vi "UHR-Fleezers Control (host) - 10.8MV_trial1.vi"() -> ()   [LabVIEW 2010] (continued)
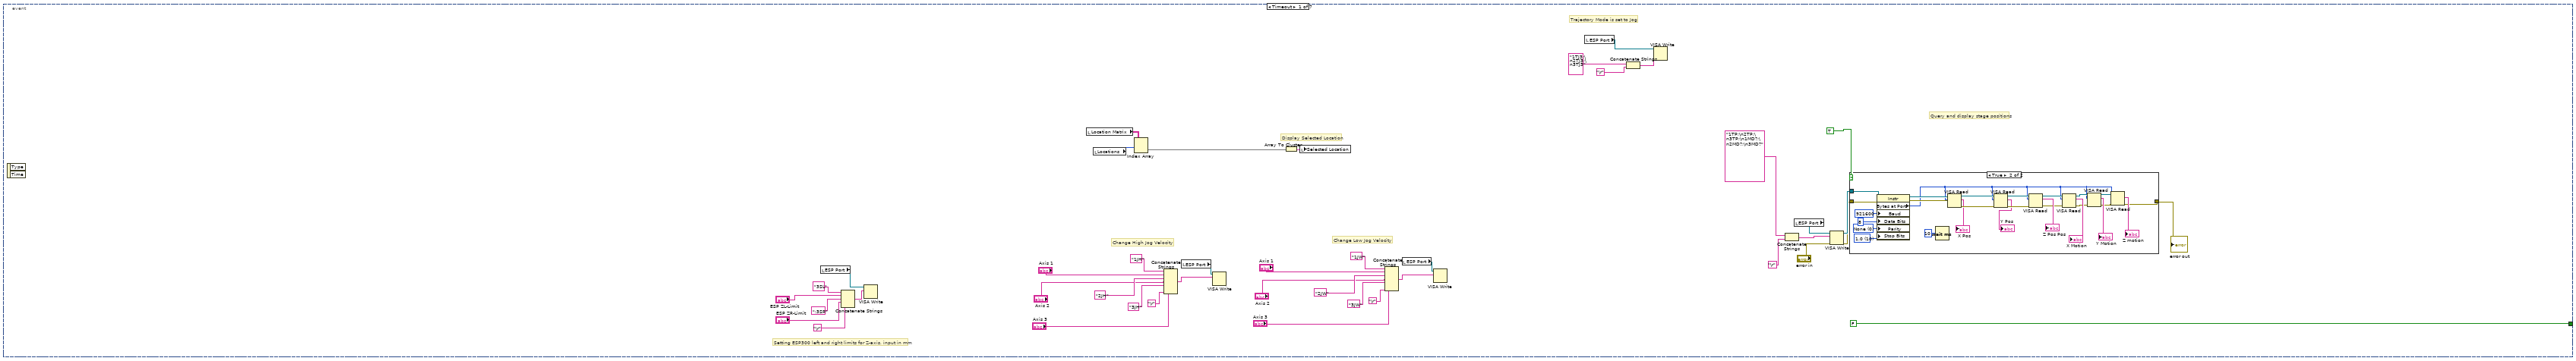
[diagram p2: hidden frame]
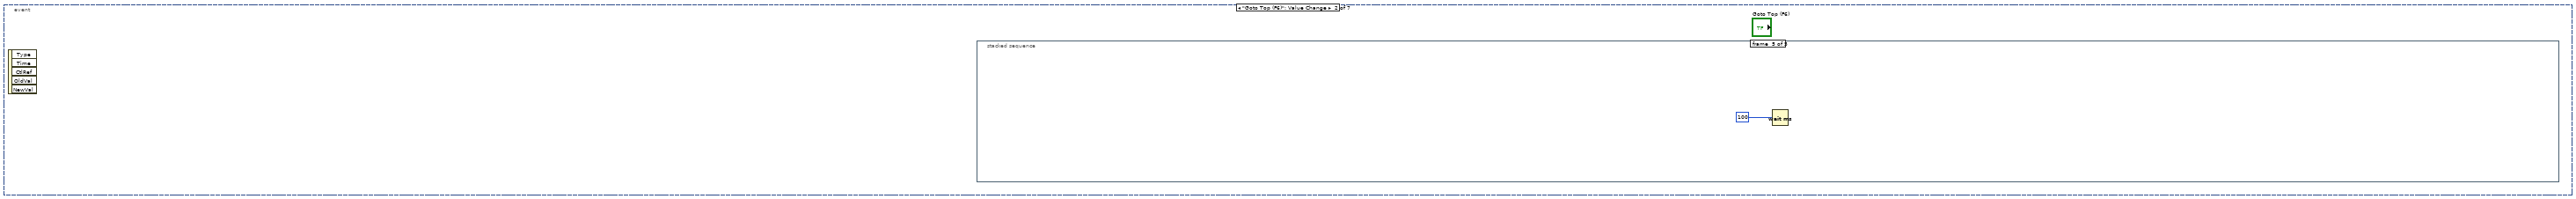
[diagram p4: hidden frame]
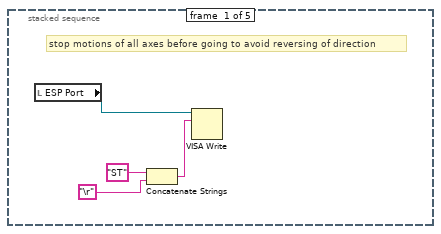
[diagram p5: hidden frame]
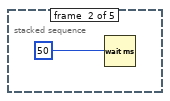
[diagram p6: hidden frame]
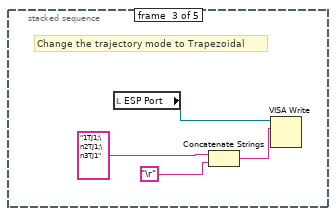
[diagram p7: hidden frame]
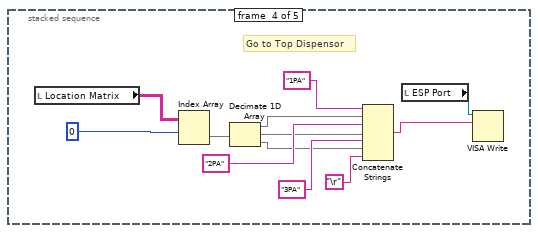
[diagram p8: hidden frame]
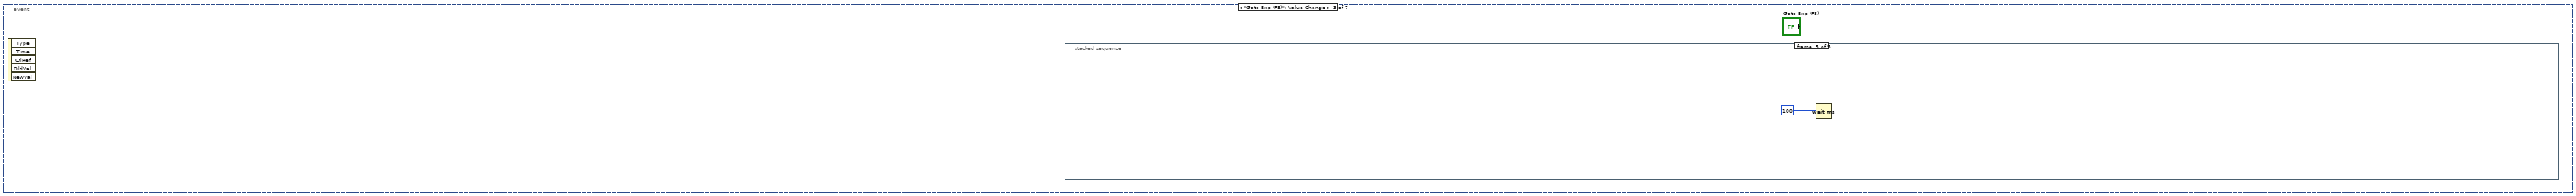
[diagram p9: hidden frame]
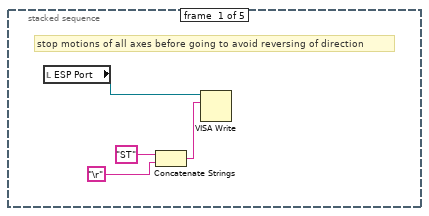
[diagram p10: hidden frame]
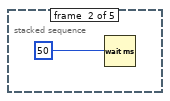
[diagram p11: hidden frame]
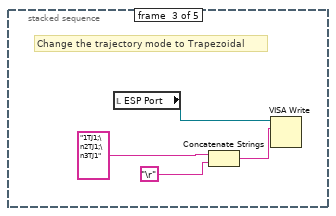
[diagram p12: hidden frame]
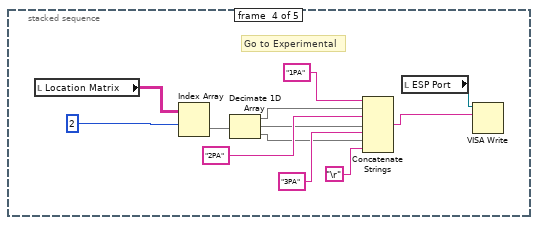
[diagram p13: hidden frame]
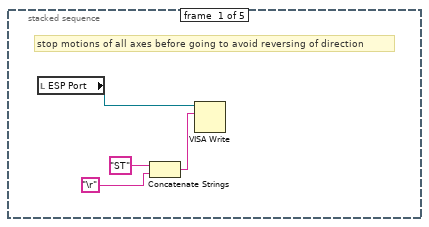
[diagram p14: hidden frame]
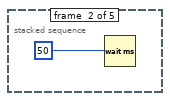
[diagram p15: hidden frame]
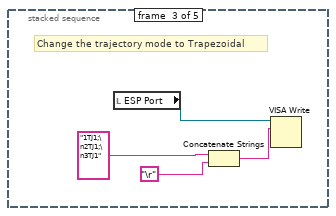
[diagram p16: hidden frame]
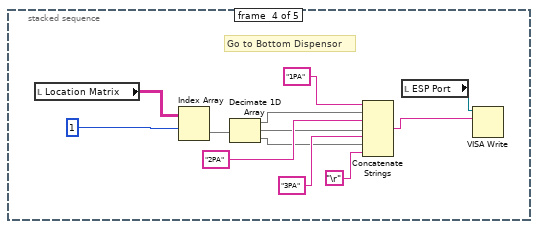
[diagram p17: hidden frame]
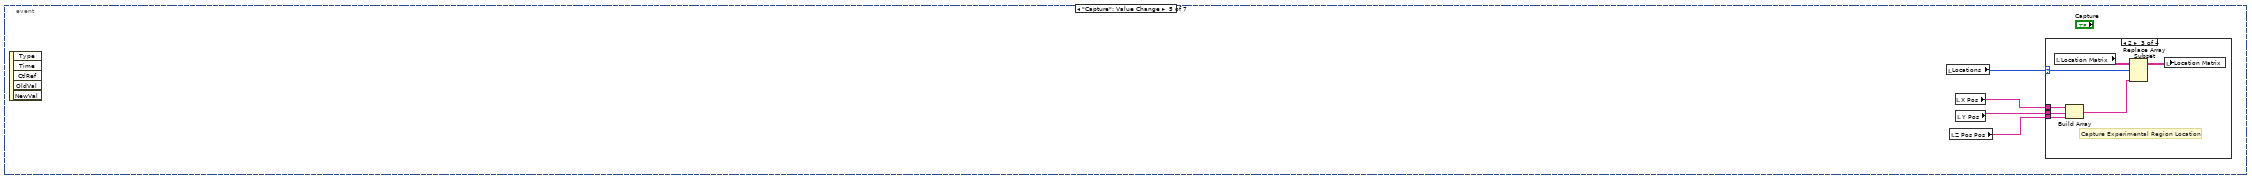
[diagram p18: hidden frame]
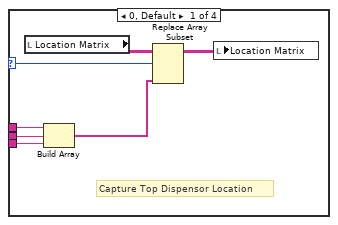
[diagram p19: hidden frame]
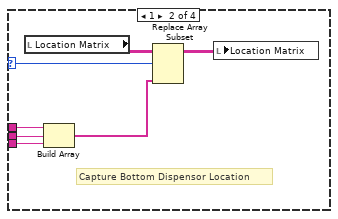
[diagram p20: hidden frame]
                n1978 = case shown="True" w8552 {
                  tunnel: w8553 -> [_ w8557]
                  frame False {
                  }
                  frame True {
                    n1979 = Close File(refnum=w8557) -> ()  [unwired: 1 in, 2 out]
                  }
                }
                n1980 = case shown="True" w8550 {
                  tunnel: w8551 -> [_ w8556]
                  frame False {
                  }
                  frame True {
                    n1981 = Close File(refnum=w8556) -> ()  [unwired: 1 in, 2 out]
                  }
                }
                n1982 = local write "Calibrating Trap..."(w8549) -> ()
                n1983 = call <vilib>:"Beep.vi"() -> ()  [unwired: 3 in, 9 out]
                n1984 = local write "Stop Saving"(w8549) -> ()
                n1985 = property on="Raster Scanning..." class="Bool (strict)"("Val(Sgnl)"=w8549) -> ()  [unwired: 2 in, 2 out]
                "Saving..." <- w8549
              }
              frame True {
                n1986 = local read "Calibrating Trap..."() -> (w8615:bool)
                n1987 = case "Write fl. data" shown="True" w8614 {
                  tunnel: w8613 -> [_ w8649]
                  tunnel: w8612 -> [_ w8648]
                  frame False {
                  }
                  frame True {
                    n1988 = Write to Binary File(file (use dialog)=w8649, data=w8648, 5:FALSE ("prepend array or string size? (T)"), 9:T31."big-endian, network order" ("byte order (0:big-endian, network order)")) -> ()  [unwired: 1 in, 4 out]
                  }
                }
                n1989 = Greater?(x="Save ave N", y=1.0) -> (0:w8618:bool)
                n1990 = Not(x=w8615) -> (.not. x?=w8617:bool)
                n1991 = And(x=w8617, y=w8618) -> (x .and. y?=w8560:bool)
                n1992 = case shown="True" w8560 {
                  tunnel: w8559 -> [w8629 w8640]
                  tunnel: [w8629 w8632] -> w8558
                  tunnel: "Save ave N" -> [_ w8633]
                  frame False {
                  }
                  frame True {
                    w8630 = 2 ("dimension size")
                    n1993 = Array Size(array=w8640) -> (size(s)=w8634:i32)
                    n1994 = Divide(x=w8634, y=w8630) -> (x/y=w8638:dbl)
                    n1995 = Reshape Array(w8640, w8638, w8630) -> (w8639:u64[][])
                    n1996 = Transpose 2D Array(2D array=w8639) -> (transposed array=w8637:u64[][])
                    n1997 = for {
                      tunnel: w8637 -> [w8642] mode=indexing
                      tunnel: [w8641] -> w8631 mode=indexing
                      tunnel: w8633 -> [w8643]
                      workers-P: _ -> [_]
                      n1998 = call "downsample 1D array - U64.vi"("Ave N"=w8643, "Array In"=w8642) -> ("Array Out"=w8641:u64[])  [unwired: 1 in]
                    }
                    n1999 = Transpose 2D Array(2D array=w8631) -> (transposed array=w8636:u64[][])
                    n2000 = Divide(x=w8634, y=w8633) -> (x/y=w8635:dbl)
                    n2001 = Reshape Array(w8636, w8635) -> (w8632:u64[])
                  }
                }
                n2002 = case shown="True" w8560 {
                  tunnel: w8620 -> [w8652 w8664]
                  tunnel: [w8652 w8656] -> w8616
                  tunnel: "Save ave N" -> [_ w8657]
                  tunnel: w8611 -> [_ w8655]
                  frame False {
                    # "don't downsample data for trap calibration"
                  }
                  frame True {
                    n2003 = Array Size(array=w8664) -> (size(s)=w8658:i32)
                    n2004 = Array Size(array=w8655) -> (size(s)=w8654:i32)
                    n2005 = Divide(x=w8658, y=w8654) -> (x/y=w8662:dbl)
                    n2006 = Reshape Array(w8664, w8662, w8654) -> (w8663:i16[][])
                    n2007 = Transpose 2D Array(2D array=w8663) -> (transposed array=w8661:i16[][])
                    n2008 = for {
                      tunnel: w8661 -> [w8667] mode=indexing
                      tunnel: [w8666] -> w8653 mode=indexing
                      tunnel: w8657 -> [w8665]
                      workers-P: _ -> [_]
                      n2009 = call "downsample 1D array - I16.vi"("Ave N"=w8665, "Array In"=w8667) -> ("Array Out"=w8666:i16[])  [unwired: 1 out]
                    }
                    n2010 = Transpose 2D Array(2D array=w8653) -> (transposed array=w8660:i16[][])
                    n2011 = Divide(x=w8658, y=w8657) -> (x/y=w8659:dbl)
                    n2012 = Reshape Array(w8660, w8659) -> (w8656:i16[])
                  }
                }
                n2013 = Index Array(array=w8582, index=1) -> (element=w8585:waveform(dbl))
                n2014 = Index Array(array=w8582, index=0) -> (element=w8587:waveform(dbl))
                n2015 = Unbundle By Name(w8585) -> ("Y"=w8589:dbl[])
                n2016 = Unbundle By Name(w8587) -> ("Y"=w8597:dbl[])
                n2017 = case "Write trap pos. data" shown="True" w8563 {
                  tunnel: w8562 -> [_ w8645]
                  tunnel: w8558 -> [_ w8644]
                  frame False {
                  }
                  frame True {
                    n2018 = Write to Binary File(file (use dialog)=w8645, data=w8644, 5:FALSE ("prepend array or string size? (T)"), 9:T31."big-endian, network order" ("byte order (0:big-endian, network order)")) -> ()  [unwired: 1 in, 4 out]
                  }
                }
                n2019 = Write to Binary File(file (use dialog)=w8623, data=w8616, 5:FALSE ("prepend array or string size? (T)"), 9:T31."big-endian, network order" ("byte order (0:big-endian, network order)")) -> ()  [unwired: 1 in, 4 out]
                n2020 = feedback #26(w8589) -> (w8591:dbl[])
                n2021 = Build Array (concatenate)(w8591, w8589) -> (w8590:dbl[])
                n2022 = Select(t=w8589, s=w8565, f=w8590) -> (s? t:f=w8575:dbl[])
                n2023 = feedback-in #26(w8575) -> ()
                n2024 = feedback #27(w8597) -> (w8610:dbl[])
                n2025 = Build Array (concatenate)(w8610, w8597) -> (w8609:dbl[])
                n2026 = Select(t=w8597, s=w8565, f=w8609) -> (s? t:f=w8584:dbl[])
                n2027 = feedback-in #27(w8584) -> ()
                n2028 = Divide(x=w8624, y=w8625) -> (x/y=w8627:dbl)
                n2029 = Multiply(x=w8627, y=100.0) -> (x*y=w8626:dbl)
                n2030 = Build Array(w8584, w8575) -> (→"Saved APD":dbl[][])
                n2031 = Array Size(array=w8584) -> (size(s)=w8602:i32)
                n2032 = Unbundle By Name(w8604) -> ("Y"=w8608:dbl[])
                n2033 = Subtract(x=w8602, y="N pts to average") -> (x-y=w8578:i32)
                n2034 = Multiply(x="N pts to average", y=u16 2) -> (x*y=w8579:u16)
                n2035 = Subtract(x=w8602, y=w8579) -> (x-y=w8577:i32)
                n2036 = feedback #28(w8608) -> (w8607:dbl[])
                n2037 = Build Array (concatenate)(w8607, w8608) -> (w8606:dbl[])
                n2038 = Select(t=w8608, s=w8565, f=w8606) -> (s? t:f=w8605:dbl[])
                "Trap Delta Graph" <- w8605
                n2039 = feedback-in #28(w8605) -> ()
                n2040 = Array Subset(array=w8584, index=w8578, length="N pts to average") -> (w8601:dbl[])
                n2041 = Array Subset(array=w8584, index=w8577, length="N pts to average") -> (w8600:dbl[])
                n2042 = Array Subset(array=w8575, index=w8578, length="N pts to average") -> (w8581:dbl[])
                n2043 = Array Subset(array=w8575, index=w8577, length="N pts to average") -> (w8580:dbl[])
                n2044 = call <vilib>:"Mean.vi"("X"=w8601) -> ("mean"=w8599:dbl)  [unwired: 1 out]
                n2045 = call <vilib>:"Mean.vi"("X"=w8581) -> ("mean"=w8574:dbl)  [unwired: 1 out]
                n2046 = call <vilib>:"Mean.vi"("X"=w8600) -> ("mean"=w8598:dbl)  [unwired: 1 out]
                n2047 = call <vilib>:"Mean.vi"("X"=w8580) -> ("mean"=w8573:dbl)  [unwired: 1 out]
                n2048 = Subtract(x=w8574, y=w8573) -> (x-y=w8564:dbl)
                "Delta Fl. 2" <- w8564
                n2049 = Subtract(x=w8599, y=w8598) -> (x-y=w8596:dbl)
                "Delta Fl. 1" <- w8596
                n2050 = Initialize Array(w8596, 1 ("dimension size")) -> (w8593:dbl[])
                n2051 = Initialize Array(w8564, 1 ("dimension size")) -> (w8570:dbl[])
                n2052 = feedback #29(w8593) -> (w8594:dbl[])
                n2053 = Build Array (concatenate)(w8594, w8593) -> (w8592:dbl[])
                n2054 = feedback #30(w8570) -> (w8571:dbl[])
                n2055 = Build Array (concatenate)(w8571, w8570) -> (w8569:dbl[])
                n2056 = Select(t=w8593, s=w8565, f=w8592) -> (s? t:f=w8568:dbl[])
                n2057 = feedback-in #29(w8568) -> ()
                n2058 = Select(t=w8570, s=w8565, f=w8569) -> (s? t:f=w8567:dbl[])
                n2059 = feedback-in #30(w8567) -> ()
                n2060 = Build Array(w8568, w8567) -> (→"Save APD Deriv":dbl[][])
              }
            }
            "Progress" <- w8541
            "Progress 2" <- w8541
          }
        }
      }
    }
    n2061 = Bundle By Name(cluster=w5584, "Green FB Ch 0"=w5583, "Green FB Ch 1"=w5582) -> (w5562:T50)
    "Green FB Signals (V)" <- w5562
    n2062 = Unbundle By Name(w5562) -> ("Green FB Ch 2"=→"Green FB Plot":dbl)
    n2063 = local read "wait to reset values"() -> (w5654:bool)
    n2064 = Not(x=w5651) -> (.not. x?=w5655:bool)
    n2065 = And(x=w5655, y=w5654) -> (x .and. y?=w5656:bool)
    n2066 = case "Part of MCL raster scanning: returns to initial positions after scan done" shown="True" w5656 {
      tunnel: w5659 -> [w7258 w7265]
      tunnel: [w7258 w7264] -> w5658
      tunnel: w5653 -> [w7257 w7263]
      tunnel: [w7257 w7262] -> w5652
      frame False {
      }
      frame True {
        w7273 = 10.0 ("y")
        w7272 = 32767.0 ("y")
        # "to return scan values\nafter a synchronous \nAOM scan"
        n2067 = local read "AO2"() -> (w7266:dbl)
        n2068 = local read "AO1"() -> (w7267:dbl)
        n2069 = local write "wait to reset values"(FALSE ("wait to reset values")) -> ()
        n2070 = Multiply(x=w7267, y=w7272) -> (x*y=w7269:dbl)
        n2071 = Multiply(x=w7266, y=w7272) -> (x*y=w7271:dbl)
        n2072 = Divide(x=w7269, y=w7273) -> (x/y=w7268:dbl)
        n2073 = Divide(x=w7271, y=w7273) -> (x/y=w7270:dbl)
        n2074 = To Word Integer(number=w7268) -> (16bit integer=w7274:i16)
        n2075 = To Word Integer(number=w7270) -> (16bit integer=w7275:i16)
        n2076 = local read "Total Counts (ticks)"() -> (w7259:u32)
        n2077 = xnode "Read/Write Control"("FPGA VI Reference In"=w7265, "error in"=w7263, "AO1"=w7274, "AO2"=w7275, "MCL count"=w7259) -> ("FPGA VI Reference Out"=w7264:T19, "error out"=w7262:errorcluster)
        n2078 = local read "Scan Range (V)\n(of steps)"() -> (w7260:dbl)
        n2079 = property on="Scan Range (V)\n(of steps)" class="DigNum (strict)"("Val(Sgnl)"=w7260) -> ()  [unwired: 2 in, 2 out]
      }
    }
    n2080 = node-c288() -> ()  [unwired: 2 out]
  }
  n2081 = node-c288(3 ("Processor")) -> (w74:T26)  [unwired: 3 out]
  n2082 = timed-loop "Oscillate AOD (debugging)" {
    tunnel: w24 -> [w8669]
    tunnel: [w8668] -> w36
    timing: w74 -> [_]
    timing-out: [_] -> w73
    stop <- w8668 stop-if-true
    n2083 = node-c288() -> ()  [unwired: 2 out]
    n2084 = event shown="[0] \"Oscillate Set 2\", \"Fish for Tether\": Value Change" {
      selector: _ -> [_ _ _]
      dyn-events: _ -> [_ _ _]
      timeout: _ -> [_ _ _]
      tunnel: w8669 -> [w8676 _ _]
      tunnel: [FALSE ("Stop All") _ w8944] -> w8668
      event "Oscillate Set 2", "Fish for Tether": Value Change {
        n2085 = event-data() -> ()  [unwired: 6 out]
        n2086 = local read "Oscillate Set 2"() -> (w8675:bool)
        n2087 = Or(x=w8675, y="Fish for Tether") -> (x .or. y?=w8673:bool)
        n2088 = case shown="True" w8673 {
          tunnel: w8676 -> [_ w8679]
          tunnel: "Fish for Tether" -> [_ w8678]
          frame False {
          }
          frame True {
            n2089 = case shown="True" w8678 {
              frame False {
              }
              frame True {
                n2090 = local write "Scan axis 2"(TRUE) -> ()
                n2091 = local write "Tether"(FALSE ("Tether")) -> ()
              }
            }
            n2092 = node-c288("Period") -> (w8681:T26)  [unwired: 3 out]
            n2093 = timed-loop "Oscillate AOD" {
              timing: w8681 -> [_]
              timing-out: [_] -> w8680
              tunnel: w8679 -> [w8691]
              tunnel: w8678 -> [w8690]
              i -> [w8693]
              stop <- w8689 stop-if-true
              n2094 = node-c288() -> (w8692:i64)  [unwired: 1 out]
              n2095 = flat-sequence {
                tunnel: w8693 -> [w8719]
                tunnel: w8692 -> [w8718]
                tunnel: w8691 -> [w8702]
                tunnel: w8690 -> [w8704]
                tunnel: [w8704] -> w8688
                tunnel: [w8703] -> w8687
                tunnel: [w8701] -> w8686
                tunnel: [w8698] -> w8684
                tunnel: w8688 -> [w8755]
                tunnel: w8687 -> [w8753]
                tunnel: w8686 -> [w8752]
                tunnel: [w8751] -> w8685
                tunnel: w8684 -> [w8750]
                tunnel: [w8819] -> w8689
                tunnel: w8685 -> [w8817]
                frame #0 {
                  n2096 = Divide(x=w8718, y=i64 1000) -> (x/y=w8713:dbl)
                  n2097 = Multiply(x=w8713, y=w8719) -> (x*y=w8715:dbl)
                  n2098 = Multiply(x="Osc. freq. (Hz)", y=6.283185307179586) -> (x*y=w8716:dbl)
                  n2099 = Multiply(x=w8716, y=w8715) -> (x*y=w8700:dbl)
                  n2100 = local read "BD 1 Frequency 2 (MHz)"() -> (w8697:dbl)
                  n2101 = local read "BD 1 Frequency 1 (MHz)"() -> (w8694:dbl)
                  n2102 = case shown="True" w8704 {
                    tunnel: w8700 -> [w8725 w8732]
                    tunnel: w8697 -> [_ w8742]
                    tunnel: [w8722 w8726] -> w8705
                    tunnel: [FALSE w8735] -> w8701
                    tunnel: [0.0 w8728] -> w8698
                    tunnel: w8694 -> [_ w8727]
                    frame False {
                      n2103 = Sine(x=w8725) -> (sin(x)=w8723:dbl)
                      n2104 = Multiply(x=w8723, y="Osc. amp. (MHz)") -> (x*y=w8722:dbl)
                    }
                    frame True {
                      n2105 = Cosine(x=w8732) -> (cos(x)=w8745:dbl)
                      n2106 = Subtract(x=w8742, y=w8727) -> (x-y=w8741:dbl)
                      n2107 = Decrement(x=w8745) -> (x-1=w8744:dbl)
                      n2108 = Subtract(x=w8741, y="Closest Delta (MHz)") -> (x-y=w8738:dbl)
                      n2109 = Divide(x=w8744, y=2.0) -> (x/y=w8739:dbl)
                      n2110 = Multiply(x=w8739, y=w8738) -> (x*y=w8726:dbl)
                      n2111 = local read "Vec Mean of T1 T2"() -> (w8734:dbl[])
                      n2112 = Greater?(x=w8734, y="Stop F (pN)") -> (0:w8736:bool[])
                      n2113 = Or Array Elements(Boolean array=w8736) -> (logical OR=w8735:bool)
                      n2114 = Divide(x=w8732, y=6.283185307179586) -> (x/y=w8731:dbl)
                      n2115 = Round Toward +Infinity(x=w8731) -> (ceil(x): smallest int >= x=w8728:dbl)
                      "Attempts" <- w8728
                      n2116 = Greater?(x=w8728, y="Attempt Limit") -> (0:w8730:bool)
                      n2117 = case shown="True" w8730 {
                        frame False {
                        }
                        frame True {
                          n2118 = local write "Fish for Tether"(FALSE ("Fish for Tether")) -> ()
                          n2119 = call <vilib>:"Beep.vi"() -> ()  [unwired: 3 in, 9 out]
                          n2120 = local read "Messages"() -> (w8747:string)
                          n2121 = call "Update messages.vi"("Message to add"="Tether fishing timeout." ("Messages"), "Old message string"=w8747) -> ("New message string"=→"Messages":string)
                        }
                      }
                    }
                  }
                  n2122 = local read "Y RF Frequency Limits (MHz)"() -> (w8706:T16)
                  n2123 = local read "X RF Frequency Limits (MHz)"() -> (w8707:T16)
                  n2124 = local read "BD 1 Frequency 3 (MHz)"() -> (w8712:dbl)
                  n2125 = local read "BD 2 Frequency 2 (MHz)"() -> (w8696:dbl)
                  n2126 = Select(t=w8697, s="Scan axis 2", f=w8696) -> (s? t:f=w8708:dbl)
                  n2127 = Add(x=w8705, y=w8708) -> (x+y=w8703:dbl)
                  n2128 = Select(t=w8703, s="Scan axis 2", f=w8697) -> (s? t:f=w8695:dbl)
                  n2129 = Select(t=w8696, s="Scan axis 2", f=w8703) -> (s? t:f=w8710:dbl)
                  n2130 = local read "BD 2 Frequency 3 (MHz)"() -> (w8711:dbl)
                  n2131 = call "set RF board frequency - interlace.vi"("Board 2 Frequency Limits"=w8706, "Board 1 Frequency Limits"=w8707, "FPGA VI Reference In"=w8702, "Board 2 Frequency 3 (MHz)"=w8711, "Board 1 Frequency 3 (MHz)"=w8712, "Board 2 Frequency 2 (MHz)"=w8696, "Board 2 Frequency 1 (MHz)"=w8710, "Board 1 Frequency 2 (MHz)"=w8695, "Board 1 Frequency 1  (MHz)"=w8694) -> ()  [unwired: 1 in, 2 out]
                }
                frame #1 {
                  n2132 = And(x=w8755, y=w8752) -> (x .and. y?=w8754:bool)
                  n2133 = case "Only if were fishing and now formed tether" shown="True" w8754 {
                    tunnel: w8753 -> [w8757 w8769]
                    tunnel: [w8756 w8768] -> w8751
                    tunnel: w8750 -> [_ w8764]
                    frame False {
                      n2134 = local read "Fish for Tether"() -> (w8756:bool)
                      n2135 = case shown="True" w8756 {
                        tunnel: w8757 -> [_ _]
                        frame False {
                        }
                        frame True {
                        }
                      }
                    }
                    frame True {
                      w8768 = FALSE ("Fish for Tether")
                      n2136 = call <vilib>:"Beep.vi"() -> ()  [unwired: 3 in, 9 out]
                      n2137 = Number To Decimal String(number=w8764, width (-)=i16 1) -> (decimal integer string=w8762:string)
                      n2138 = case shown="\"2\", \"3\", \"4\", \"5\", \"6\"" "Then..." {
                        selector: "Then..." -> [_ w8772]
                        tunnel: w8769 -> [w8771 _]
                        frame "1", Default {
                          # "do nothing"
                          n2139 = property on="BD 1 Frequency 1 (MHz)" class="DigNum (strict)"("Val(Sgnl)"=w8771) -> ()  [unwired: 2 in, 2 out]
                        }
                        frame "2", "3", "4", "5", "6" {
                          n2140 = flat-sequence {
                            tunnel: w8772 -> [w8774]
                            frame #0 {
                              n2141 = property on="Trap Delta (MHz)" class="DigNum (strict)"("Val(Sgnl)"="Move to Delta 1 (MHz)") -> ()  [unwired: 2 in, 2 out]
                            }
                            frame #1 {
                              n2142 = case shown="\"5\", \"6\"" w8774 {
                                selector: w8774 -> [w8777 w8787 _]
                                frame "3", "4" {
                                n2143 = flat-sequence {
                                tunnel: w8777 -> [w8778]
                                tunnel: [w8778] -> w8775
                                tunnel: [w8780] -> w8776
                                tunnel: w8775 -> [w8780]
                                tunnel: w8776 -> [w8784]
                                frame #0 {
                                n2144 = property on="Green Laser ON/Interlacing" class="Bool (strict)"("Val(Sgnl)"=TRUE ("Value (Signaling)")) -> ()  [unwired: 2 in, 2 out]
                                }
                                frame #1 {
                                n2145 = Multiply(x="Wait Before Save (s)", y=u32 1000 ("x")) -> (x*y=w8782:u32)
                                n2146 = Wait (ms)(milliseconds to wait=w8782) -> ()  [unwired: 1 out]
                                }
                                frame #2 {
                                n2147 = property on="Start Saving" class="Bool (strict)"("Value"=TRUE ("Start Saving")) -> ()  [unwired: 2 in, 2 out]
                                n2148 = case shown="Default" w8784 {
                                frame Default {
                                }
                                frame "4" {
                                n2149 = property on="Fl. Triggered..." class="Bool (strict)"("Val(Sgnl)"=TRUE ("Value (Signaling)")) -> ()  [unwired: 2 in, 2 out]
                                }
                                }
                                }
                                }
                                }
                                frame "5", "6" {
                                n2150 = stacked-sequence {
                                tunnel: w8787 -> [_ _ _ _ _ _ _ _ w8804 _ _]
                                frame #0 {
                                n2151 = Replace Array Subset(array=u32[] [0] ("Index Values"), new element="Raster Set Upon Tether", index=0) -> (w8788:u32[])
                                n2152 = property on="Saved AOD Raster Scan Parameter Sets" class="Arr (strict)"("Index Values"=w8788) -> ()  [unwired: 2 in, 2 out]
                                }
                                frame #1 {
                                n2153 = Wait (ms)(milliseconds to wait=u32 500) -> ()  [unwired: 1 out]
                                }
                                frame #2 {
                                n2154 = property on="Load parameters" class="Bool (strict)"("Val(Sgnl)"=TRUE ("Value (Signaling)")) -> ()  [unwired: 2 in, 2 out]
                                }
                                frame #3 {
                                n2155 = Wait (ms)(milliseconds to wait=u32 500) -> ()  [unwired: 1 out]
                                }
                                frame #4 {
                                n2156 = property on="Trap Raster Scan" class="Bool (strict)"("Val(Sgnl)"=TRUE ("Value (Signaling)")) -> ()  [unwired: 2 in, 2 out]
                                }
                                frame #5 {
                                n2157 = Wait (ms)(milliseconds to wait=u32 2000) -> ()  [unwired: 1 out]
                                }
                                frame #6 {
                                n2158 = while {
                                stop <- w8799 stop-if-true
                                n2159 = local read "Raster Scanning..."() -> (w8798:bool)
                                n2160 = local read "Saving..."() -> (w8801:bool)
                                n2161 = Wait (ms)(milliseconds to wait=u32 100) -> ()  [unwired: 1 out]
                                n2162 = Not(x=w8801) -> (.not. x?=w8800:bool)
                                n2163 = Not(x=w8798) -> (.not. x?=w8797:bool)
                                n2164 = And(x=w8800, y=w8797) -> (x .and. y?=w8799:bool)
                                }
                                }
                                frame #7 {
                                n2165 = property on="Trap Delta (MHz)" class="DigNum (strict)"("Val(Sgnl)"="Move to Delta 2 (MHz)") -> ()  [unwired: 2 in, 2 out]
                                }
                                frame #8 {
                                n2166 = local read "Tether"() -> (w8805:bool)
                                n2167 = case shown="True" w8805 {
                                tunnel: w8804 -> [_ w8806]
                                frame False {
                                }
                                frame True {
                                n2168 = flat-sequence {
                                tunnel: w8806 -> [w8808]
                                frame #0 {
                                n2169 = Wait (ms)(milliseconds to wait=u32 500) -> ()  [unwired: 1 out]
                                }
                                frame #1 {
                                n2170 = case shown="\"6\"" w8808 {
                                frame Default {
                                }
                                frame "6" {
                                n2171 = property on="Green Laser ON/Interlacing" class="Bool (strict)"("Val(Sgnl)"=TRUE ("Green Laser ON/Interlacing")) -> ()  [unwired: 2 in, 2 out]
                                }
                                }
                                }
                                frame #2 {
                                n2172 = Wait (ms)(milliseconds to wait=u32 500) -> ()  [unwired: 1 out]
                                }
                                frame #3 {
                                n2173 = local write "Start Saving"("Save at end (5, 6)") -> ()
                                }
                                }
                                }
                                }
                                }
                                frame #9 {
                                n2174 = local read "Bead Sep. Int. Time (s)"() -> (w8814:dbl)
                                n2175 = Multiply(x=w8814, y=1000.0) -> (x*y=w8813:dbl)
                                n2176 = Wait (ms)(milliseconds to wait=w8813) -> ()  [unwired: 1 out]
                                }
                                frame #10 {
                                n2177 = property on="Rescale on Mean" class="Bool (strict)"("Val(Sgnl)"=TRUE ("Value (Signaling)")) -> ()  [unwired: 2 in, 2 out]
                                }
                                }
                                }
                                frame "2", Default {
                                }
                              }
                            }
                          }
                        }
                      }
                      n2178 = Concatenate Strings("Formed tether in ", w8762, " attempt(s)." ("string")) -> (w8759:string)
                      n2179 = local read "Messages"() -> (w8766:string)
                      n2180 = local write "Fish for Tether"(w8768) -> ()
                      n2181 = call "Update messages.vi"("Message to add"=w8759, "Old message string"=w8766) -> ("New message string"=w8765:string)
                      n2182 = local write "Messages"(w8765) -> ()
                      n2183 = Get Date/Time In Seconds() -> (seconds since 1Jan1904=→"Time tether formed":timestamp)
                      "Tether" <- "Tether Alarm?"
                    }
                  }
                }
                frame #2 {
                  n2184 = local read "Oscillate Set 2"() -> (w8818:bool)
                  n2185 = local read "Stop All"() -> (w8820:bool)
                  n2186 = Not Or(1:w8817, 2:w8818) -> (0:w8816:bool)
                  n2187 = Compound Arithmetic op=OR(w8820, w8816) -> (w8819:bool)
                }
              }
              n2188 = node-c288() -> ()  [unwired: 2 out]
            }
            n2189 = node-c288(w8680) -> ()  [unwired: 1 out]
          }
        }
      }
      event "Fl. Triggered...": Value Change {
        n2190 = event-data() -> ()  [unwired: 7 out]
        n2191 = case shown="True" "Fl. Triggered..." {
          frame False {
          }
          frame True {
            n2192 = node-c288() -> (w8832:T26)  [unwired: 4 out]
            n2193 = timed-loop {
              timing: w8832 -> [_]
              timing-out: [_] -> w8831
              tunnel: "Action" -> [w8836]
              shift-right: [w8833] -> _
              shift-left: u8 255 -> [w8835]
              stop <- w8837 stop-if-true
              n2194 = node-c288() -> ()  [unwired: 2 out]
              n2195 = flat-sequence {
                tunnel: w8836 -> [w8849]
                tunnel: w8835 -> [w8846]
                tunnel: [w8845] -> w8834
                tunnel: [w8935] -> w8837
                tunnel: w8834 -> [w8934]
                tunnel: [w8934] -> w8833
                frame #0 {
                  n2196 = local read "Delta Fl. 2"() -> (w8840:dbl)
                  n2197 = local read "Delta Fl. 1"() -> (w8841:dbl)
                  n2198 = Select(t=w8841, s="APD to Watch", f=w8840) -> (s? t:f=w8839:dbl)
                  n2199 = Multiply(x="Fl. Delta Thresh. (kHz)", y=1000.0) -> (x*y=w8848:dbl)
                  n2200 = Greater?(x=w8839, y=w8848) -> (0:w8843:bool)
                  n2201 = Or(x="Force Yank", y=w8843) -> (x .or. y?=w8844:bool)
                  n2202 = case shown="True" w8844 {
                    tunnel: w8849 -> [_ w8859]
                    tunnel: w8846 -> [w8851 w8855]
                    tunnel: [w8851 w8852] -> w8845
                    frame False {
                    }
                    frame True {
                      n2203 = flat-sequence {
                        tunnel: w8856 -> [w8865]
                        tunnel: [w8865] -> w8860
                        tunnel: w8859 -> [w8864]
                        tunnel: [w8864] -> w8858
                        tunnel: [w8863] -> w8857
                        tunnel: w8855 -> [w8862]
                        tunnel: [w8861] -> w8854
                        tunnel: w8860 -> [w8890]
                        tunnel: w8858 -> [w8889]
                        tunnel: w8857 -> [w8888]
                        tunnel: w8854 -> [w8887]
                        tunnel: [w8887] -> w8853
                        tunnel: w8853 -> [w8932]
                        tunnel: [w8932] -> w8852
                        frame #0 {
                          n2204 = call <vilib>:"Beep.vi"() -> ()  [unwired: 3 in, 9 out]
                          n2205 = local write "Waiting"(FALSE ("Waiting")) -> ()
                          n2206 = Increment(x=w8862) -> (x+1=w8861:u8)
                          n2207 = case shown="\"Yank\"" w8864 {
                            tunnel: w8861 -> [_ _ w8871]
                            frame "Image" {
                              n2208 = property on="Confocal Image" class="Bool (strict)"("Val(Sgnl)"=TRUE ("Value (Signaling)")) -> ()  [unwired: 2 in, 2 out]
                            }
                            frame "Alarm", Default {
                            }
                            frame "Yank" {
                              n2209 = flat-sequence {
                                tunnel: w8871 -> [w8874]
                                tunnel: [w8873] -> w8870
                                tunnel: ["N Array El"] -> w8869
                                tunnel: w8870 -> [w8884]
                                tunnel: w8869 -> [w8880]
                                frame #0 {
                                n2210 = Multiply(x="Yank Delay (s)", y=1000.0) -> (x*y=w8877:dbl)
                                n2211 = Quotient & Remainder(x=w8874, y="N Array El") -> (x-y*floor(x/y)=w8873:u8)  [unwired: 1 out]
                                n2212 = Wait (ms)(milliseconds to wait=w8877) -> ()  [unwired: 1 out]
                                }
                                frame #1 {
                                n2213 = Random Number (0-1)() -> (number: 0 to 1=w8881:dbl)
                                n2214 = Multiply(x=w8880, y=w8881) -> (x*y=w8879:dbl)
                                n2215 = Round Toward -Infinity(1:w8879) -> (0:w8878:dbl)
                                n2216 = Select(t=w8878, s="Random Choice", f=w8884) -> (s? t:f=w8882:dbl)
                                n2217 = Index Array(array="Yank to Delta Array (MHz)", index=w8882) -> (element=w8885:dbl)
                                n2218 = property on="Trap Delta (MHz)" class="DigNum (strict)"("Val(Sgnl)"=w8885) -> ()  [unwired: 2 in, 2 out]
                                }
                              }
                            }
                          }
                          n2219 = local read "Time (s)"() -> (w8863:dbl)
                          "Fl. High" <- TRUE ("Yanking")
                        }
                        frame #1 {
                          n2220 = node-c288() -> (w8892:T26)  [unwired: 4 out]
                          n2221 = timed-loop {
                            timing: w8892 -> [_]
                            timing-out: [_] -> w8891
                            tunnel: w8890 -> [w8908]
                            tunnel: w8889 -> [w8906]
                            tunnel: w8888 -> [w8905]
                            stop <- w8907 stop-if-true
                            n2222 = node-c288() -> ()  [unwired: 2 out]
                            n2223 = local read "Fl. Delta Thresh. (kHz)"() -> (w8900:dbl)
                            n2224 = local read "Fl. Triggered..."() -> (w8909:bool)
                            n2225 = local read "Delta Fl. 1"() -> (w8896:dbl)
                            n2226 = local read "Delta Fl. 2"() -> (w8894:dbl)
                            n2227 = local read "Stop All"() -> (w8903:bool)
                            n2228 = local read "APD to Watch"() -> (w8895:bool)
                            n2229 = Select(t=w8896, s=w8895, f=w8894) -> (s? t:f=w8893:dbl)
                            n2230 = Not(x=w8909) -> (.not. x?=w8904:bool)
                            n2231 = Multiply(x=w8900, y=1000.0) -> (x*y=w8899:dbl)
                            n2232 = Negate(x=w8899) -> (-x=w8898:dbl)
                            n2233 = Less?(x=w8893, y=w8898) -> (x < y?=w8902:bool)
                            n2234 = Compound Arithmetic op=OR(w8902, w8903, w8904, "Force Reset") -> (w8907:bool)
                            n2235 = case shown="True" w8907 {
                              tunnel: w8908 -> [_ w8920]
                              tunnel: w8906 -> [_ w8919]
                              tunnel: w8905 -> [_ w8917]
                              frame False {
                              }
                              frame True {
                                n2236 = case shown="\"Yank\"" w8919 {
                                tunnel: w8920 -> [_ w8921]
                                frame "Image", Default {
                                }
                                frame "Yank" {
                                n2237 = flat-sequence {
                                tunnel: [w8926] -> w8922
                                tunnel: w8921 -> [w8926]
                                tunnel: w8922 -> [w8927]
                                frame #0 {
                                n2238 = local read "Yank Delay (s)"() -> (w8925:dbl)
                                n2239 = Multiply(x=w8925, y=1000.0) -> (x*y=w8923:dbl)
                                n2240 = Wait (ms)(milliseconds to wait=w8923) -> ()  [unwired: 1 out]
                                }
                                frame #1 {
                                n2241 = property on="Trap Delta (MHz)" class="DigNum (strict)"("Val(Sgnl)"=w8927) -> ()  [unwired: 2 in, 2 out]
                                }
                                }
                                }
                                }
                                n2242 = local read "Time (s)"() -> (w8918:dbl)
                                n2243 = Subtract(x=w8918, y=w8917) -> (x-y=w8914:dbl)
                                "Duration (s)" <- w8914
                                n2244 = Number To Decimal String(number=w8914, width (-)=i16 0) -> (decimal integer string=w8912:string)
                                n2245 = Concatenate Strings(w8912, " s fluorescence event." ("string")) -> (w8910:string)
                                n2246 = local read "Messages"() -> (w8916:string)
                                n2247 = call "Update messages.vi"("Message to add"=w8910, "Old message string"=w8916) -> ("New message string"=w8915:string)
                                n2248 = call <vilib>:"Beep.vi"() -> ()  [unwired: 3 in, 9 out]
                                n2249 = local write "Messages"(w8915) -> ()
                              }
                            }
                            n2250 = node-c288() -> ()  [unwired: 2 out]
                          }
                          n2251 = node-c288(w8891) -> ()  [unwired: 1 out]
                        }
                        frame #2 {
                          n2252 = local write "Fl. High"(FALSE ("Yanking")) -> ()
                        }
                      }
                      n2253 = local read "Trap Delta (MHz)"() -> (w8856:dbl)
                    }
                  }
                }
                frame #1 {
                  n2254 = local read "Stop All"() -> (w8938:bool)
                  n2255 = local read "Fl. Triggered..."() -> (w8936:bool)
                  n2256 = Not(x=w8936) -> (.not. x?=w8937:bool)
                  n2257 = Or(x=w8937, y=w8938) -> (x .or. y?=w8935:bool)
                  n2258 = Not(x=w8935) -> (.not. x?=→"Waiting":bool)
                }
              }
              n2259 = node-c288() -> ()  [unwired: 2 out]
            }
            n2260 = node-c288(w8831) -> ()  [unwired: 1 out]
          }
        }
      }
      event "Stop All": Value Change {
        n2261 = event-data() -> ()  [unwired: 7 out]
        n2262 = local read "Stop All"() -> (w8944:bool)
      }
    }
    n2263 = node-c288() -> ()  [unwired: 2 out]
  }
  n2264 = node-c288(w14) -> ()  [unwired: 1 out]
  n2265 = node-c288(w68) -> ()  [unwired: 1 out]
  n2266 = node-c288(w75) -> ()  [unwired: 1 out]
  n2267 = node-c288(w73) -> ()  [unwired: 1 out]
  n2268 = node-c288(w163) -> ()  [unwired: 1 out]
  n2269 = flat-sequence {
    tunnel: w33 -> [w8949]
    tunnel: [w8948] -> w39
    tunnel: [w8945] -> w38
    tunnel: w37 -> [_]
    tunnel: w36 -> [_]
    tunnel: w35 -> [_]
    tunnel: w34 -> [_]
    tunnel: w32 -> [w8946]
    tunnel: w39 -> [w9011]
    tunnel: w38 -> [w9010]
    frame #0 {
      w8947 = FALSE ("APD to FIFO")
      n2270 = xnode "Read/Write Control"("FPGA VI Reference In"=w8949, "error in"=w8946, "APD to FIFO"=w8947, "AI to FIFO"=w8947) -> ("FPGA VI Reference Out"=w8948:T19, "error out"=w8945:errorcluster)
    }
    frame #1 {
      n2271 = xnode "Invoke Method"("FPGA VI Reference In"=w9011, "error in"=w9010) -> ("FPGA VI Reference Out"=w9009:T19)  [unwired: 1 out]
      n2272 = xnode "Close FPGA VI Reference"("FPGA VI Reference In"=w9009) -> ()  [unwired: 1 in, 1 out]
    }
  }
